vi "Alt Disp.vi"(3 "Notifer In":refnum<notifier>) -> ()   [LabVIEW 2013]
doc: "Alternative display for altitude."
panel:
  out "Heading":string
  out "altitude":dbl format="%#.0f"
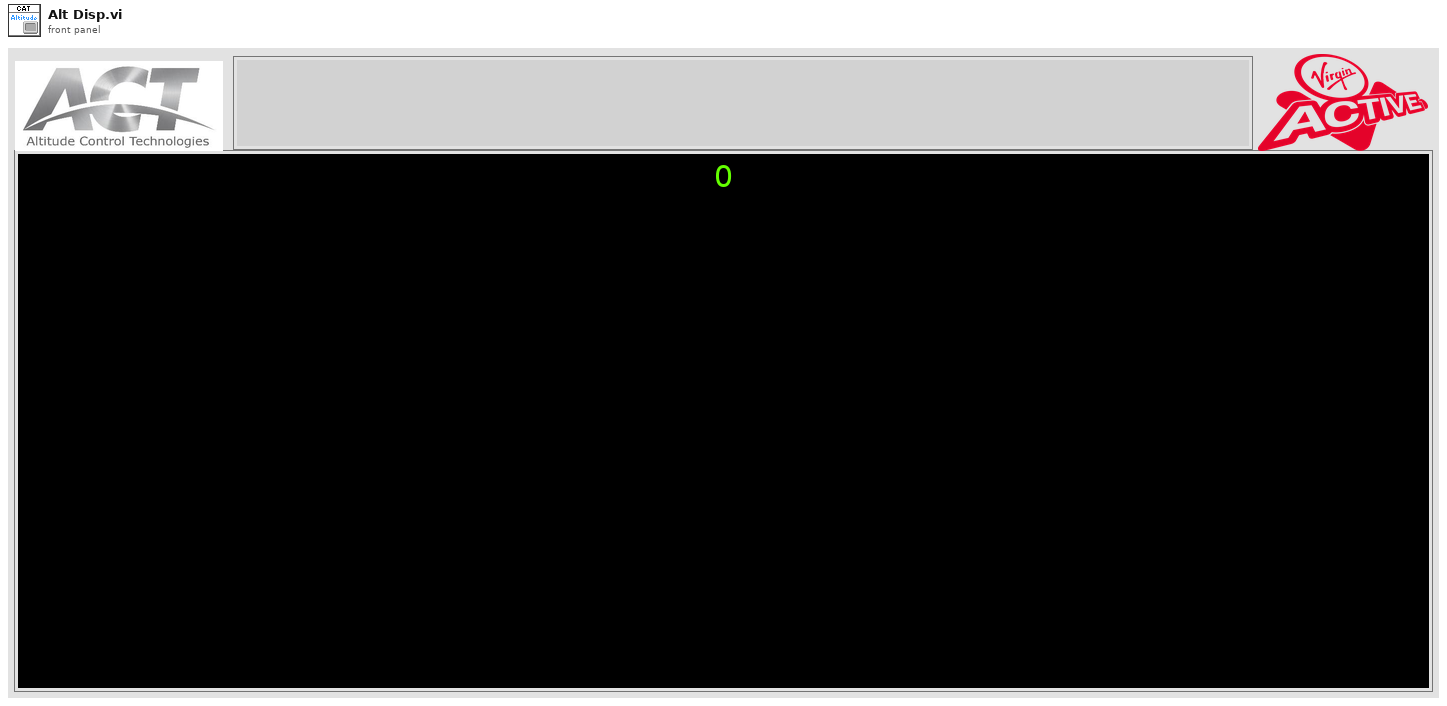
[diagram p1: front panel]
types:
  T1 = enum32{"Invalid", "Standard", "Closed", "Hidden", "Minimized", "Maximized"}
  T2 = cluster{"Heading":string, "Altitude":dbl, "Visible?":bool}
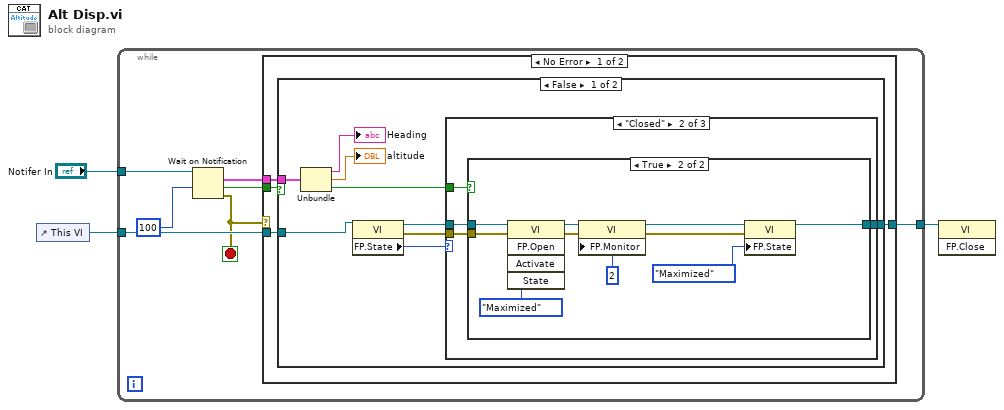
[diagram p0: block diagram]
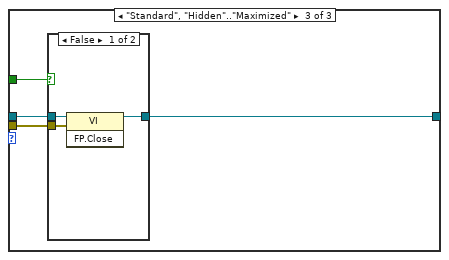
[diagram p4: hidden frame]
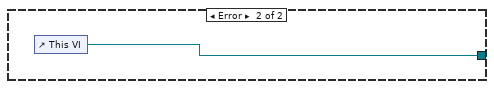
[diagram p7: hidden frame]
diagram:
  n1 = control-ref of="This VI"() -> (w1:refnum<vi>)
  n2 = while {
    tunnel: "Notifer In" -> [w10]
    tunnel: [w8] -> w2
    tunnel: w1 -> [w5]
    stop <- w4 stop-if-true
    n3 = Wait on Notification(notifier=w10, timeout in ms (-1)=100) -> (notification=w9:T2, timed out?=w6:bool, error out=w4:errorcluster)  [unwired: 2 in, 1 out]
    n4 = case shown="No Error" w4 {
      tunnel: w9 -> [w14 _]
      tunnel: [w13 w49] -> w8
      tunnel: w6 -> [w12 _]
      tunnel: w5 -> [w11 _]
      frame No Error {
        n5 = case shown="False" w12 {
          tunnel: w14 -> [w23 _]
          tunnel: [w17 w48] -> w13
          tunnel: w11 -> [w15 w48]
          frame False {
            n6 = Unbundle(w23) -> ("Heading"=→"Heading":string, "Altitude"=→"altitude":dbl, "Visible?"=w19:bool)
            n7 = property class="VI"(reference=w15) -> (reference out=w18:refnum<vi>, error out=w16:errorcluster, "FP.State"=w20:T1)  [unwired: 1 in]
            n8 = case shown="\"Closed\"" w20 {
              tunnel: w18 -> [w24 w28 w43]
              tunnel: w19 -> [_ w27 w42]
              tunnel: [w24 w26 w41] -> w17
              tunnel: w16 -> [_ w25 w40]
              frame "Invalid", Default {
              }
              frame "Closed" {
                n9 = case shown="True" w27 {
                  tunnel: w28 -> [w29 w39]
                  tunnel: [w29 w32] -> w26
                  tunnel: w25 -> [_ w35]
                  frame False {
                  }
                  frame True {
                    n10 = invoke class="VI" method="FP.Open"(reference=w39, error in=w35, "State"=T1."Maximized") -> (reference out=w37:refnum<vi>, error out=w36:errorcluster)  [unwired: 2 in, 3 out]
                    n11 = property class="VI"(reference=w37, error in=w36, "FP.Monitor"=u16 2 ("Front Panel Window:Monitor")) -> (reference out=w34:refnum<vi>, error out=w31:errorcluster)
                    n12 = property class="VI"(reference=w34, error in=w31, "FP.State"=T1."Maximized" ("Front Panel Window:State")) -> (reference out=w32:refnum<vi>)  [unwired: 1 out]
                  }
                }
              }
              frame "Standard", "Hidden".."Maximized" {
                n13 = case shown="False" w42 {
                  tunnel: w43 -> [w46 w47]
                  tunnel: [w45 w47] -> w41
                  tunnel: w40 -> [w44 _]
                  frame False {
                    n14 = invoke class="VI" method="FP.Close"(reference=w46, error in=w44) -> (reference out=w45:refnum<vi>)  [unwired: 1 in, 2 out]
                  }
                  frame True {
                  }
                }
              }
            }
          }
          frame True {
          }
        }
      }
      frame Error {
        n15 = control-ref of="This VI"() -> (w49:refnum<vi>)
      }
    }
  }
  n16 = invoke class="VI" method="FP.Close"(reference=w2) -> ()  [unwired: 2 in, 3 out]
